vi "sample F trans.vi"() -> ()   [LabVIEW 2016]
panel:
  out "Intensity Graph 12":dbl[][](graph)
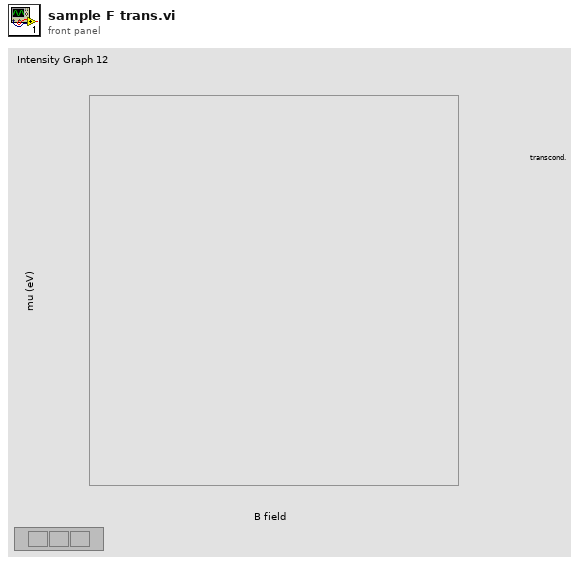
[diagram p1: front panel]
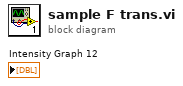
[diagram p0: block diagram]
diagram:
